vi "Dresden R2R Sputter 03.02.2018 IY24.vi"() -> ()   [LabVIEW 2009] (continued)
        n4706 = feedback #132() -> (w7120:bool)  [unwired: 1 in]
        n4707 = case shown="8" w7160 {
          tunnel: [cluster{"x":i16, "y":i16} {"x"=0, "y"=0} ("origin") cluster{"x":i16, "y":i16} {"x"=629, "y"=455} ("origin") cluster{"x":i16, "y":i16} {"x"=52, "y"=455} ("origin") cluster{"x":i16, "y":i16} {"x"=494, "y"=235} ("origin") cluster{"x":i16, "y":i16} {"x"=176, "y"=238} ("origin") cluster{"x":i16, "y":i16} {"x"=342, "y"=709} ("origin") cluster{"x":i16, "y":i16} {"x"=233, "y"=182} ("origin") cluster{"x":i16, "y":i16} {"x"=435, "y"=182} ("origin") cluster{"x":i16, "y":i16} {"x"=323, "y"=152} ("origin")] -> w7165
          tunnel: ["" ("text") "GV" ("text") "GV" ("text") "GV-BP" ("text") "GV-BP" ("text") "MG" ("text") "CST-FIX" ("text") "CST-FIX" ("text") "PET-COOL" ("text")] -> w7164
          tunnel: ["" ("DESCRIPTION") "Gate Valve" ("DESCRIPTION") "Gate Valve" ("DESCRIPTION") "Gate Valve- By Pass" ("DESCRIPTION") "Gate Valve- By Pass" ("DESCRIPTION") "MAGNETRON" ("DESCRIPTION") "Casette Fix" ("DESCRIPTION") "Casette Fix" ("DESCRIPTION") "Petfolio Cool" ("DESCRIPTION")] -> w7163
          frame #0 {
          }
          frame #1 {
          }
          frame #2 {
          }
          frame #3 {
          }
          frame #4 {
          }
          frame #5 {
          }
          frame #6 {
          }
          frame #7 {
          }
          frame #8 {
          }
        }
        n4708 = case shown="True" w7118 {
          tunnel: [TRUE FALSE] -> w7125
          tunnel: w7124 -> [_ w7209]
          frame #0 {
          }
          frame #1 {
            n4709 = call "Elapsed Time57"("Reset"=w7209) -> ("Elapsed Time (s)"=w7206:dbl)  [unwired: 11 in, 7 out]
            n4710 = Greater?(x=w7206, y=3.0) -> (0:w7207:bool)
            n4711 = In Range and Coerce(upper limit=3.0, x=w7206, lower limit=0.0) -> (In Range?=w7202:bool)  [unwired: 1 out]
            n4712 = Not(x=w7207) -> (.not. x?=w7203:bool)
            n4713 = property on="Gv_ch3_4_timer_front_gui" class="TabCtl (strict)"("Visible"=w7202) -> ()  [unwired: 2 in, 2 out]
            n4714 = local write "Gv_timer_front_ch3_4"(w7203) -> ()
          }
        }
        n4715 = case shown="True" w7093 {
          tunnel: [TRUE FALSE] -> w7122
          tunnel: w7123 -> [_ w7199]
          frame #0 {
          }
          frame #1 {
            n4716 = call "Elapsed Time58"("Reset"=w7199) -> ("Elapsed Time (s)"=w7196:dbl)  [unwired: 11 in, 7 out]
            n4717 = Greater?(x=w7196, y=3.0) -> (0:w7197:bool)
            n4718 = In Range and Coerce(upper limit=3.0, x=w7196, lower limit=0.0) -> (In Range?=w7193:bool)  [unwired: 1 out]
            n4719 = Not(x=w7197) -> (.not. x?=w7192:bool)
            n4720 = local write "Ch3_trns_gv_bp2_timer_front"(w7192) -> ()
            n4721 = property on="Ch3_trns_gv_bp2_front_gui" class="TabCtl (strict)"("Visible"=w7193) -> ()  [unwired: 2 in, 2 out]
          }
        }
        n4722 = case shown="True" w7119 {
          tunnel: [TRUE FALSE] -> w7127
          tunnel: w7126 -> [_ w7219]
          frame #0 {
          }
          frame #1 {
            n4723 = call "Elapsed Time56"("Reset"=w7219) -> ("Elapsed Time (s)"=w7216:dbl)  [unwired: 11 in, 7 out]
            n4724 = Greater?(x=w7216, y=3.0) -> (0:w7217:bool)
            n4725 = In Range and Coerce(upper limit=3.0, x=w7216, lower limit=0.0) -> (In Range?=w7212:bool)  [unwired: 1 out]
            n4726 = Not(x=w7217) -> (.not. x?=w7213:bool)
            n4727 = local write "Gv_timer_front_ch3_2"(w7213) -> ()
            n4728 = property on="Gv_ch3_2_timer_front_gui" class="TabCtl (strict)"("Visible"=w7212) -> ()  [unwired: 2 in, 2 out]
          }
        }
        n4729 = case shown="True" w7092 {
          tunnel: [TRUE FALSE] -> w7121
          tunnel: w7120 -> [_ w7189]
          frame #0 {
          }
          frame #1 {
            n4730 = call "Elapsed Time59"("Reset"=w7189) -> ("Elapsed Time (s)"=w7186:dbl)  [unwired: 11 in, 7 out]
            n4731 = Greater?(x=w7186, y=3.0) -> (0:w7187:bool)
            n4732 = In Range and Coerce(upper limit=3.0, x=w7186, lower limit=0.0) -> (In Range?=w7183:bool)  [unwired: 1 out]
            n4733 = Not(x=w7187) -> (.not. x?=w7182:bool)
            n4734 = local write "Ch3_trns_gv_bp_timer_front"(w7182) -> ()
            n4735 = property on="Ch3_trns_gv_bp_timer_front_gui" class="TabCtl (strict)"("Visible"=w7183) -> ()  [unwired: 2 in, 2 out]
          }
        }
        n4736 = local write "DESCRIPTION"(w7163) -> ()
        n4737 = call <vilib>:"Draw Text at Point.vi"("[user-specified font]"=T35 {"Font Name:"="BOLD", "Size"=18, "Strikeout?"=FALSE, "Italic?"=FALSE, "Underline?"=FALSE, "Outline?"=FALSE, "Shadow?"=FALSE, "Bold?"=TRUE} ("[user-specified font] 4"), "desired font(Application)"=T36."User-specified Font", "text"=w7164, "origin"=w7165, "picture"=w7168) -> ("new picture"=w7167:picture)  [unwired: 5 in, 1 out]
      }
    }
    "new picture 3" <- w6550
    n4738 = stacked-sequence {
      tunnel: w6559 -> [w6685 _]
      tunnel: w6560 -> [w6684 _]
      tunnel: w6561 -> [w6683 _]
      tunnel: [_ w6856] -> w6549
      tunnel: w6552 -> [w6670 _]
      tunnel: w6551 -> [w6669 _]
      tunnel: w6546 -> [w6661 _]
      tunnel: w6545 -> [w6660 _]
      tunnel: w6544 -> [w6603 _]
      tunnel: w6543 -> [w6602 _]
      tunnel: w6542 -> [w6601 _]
      tunnel: w6541 -> [w6600 _]
      tunnel: w6540 -> [w6599 _]
      tunnel: w6539 -> [w6598 _]
      tunnel: w6538 -> [w6597 _]
      tunnel: w6537 -> [w6596 _]
      tunnel: w6536 -> [w6595 _]
      tunnel: w6535 -> [w6594 _]
      tunnel: w6534 -> [w6593 _]
      tunnel: w6533 -> [w6592 _]
      tunnel: w6532 -> [w6591 _]
      tunnel: w6531 -> [w6590 _]
      tunnel: w6530 -> [w6570 _]
      tunnel: w6529 -> [w6569 _]
      frame #0 {
        n4739 = Build Array(FALSE ("element"), "chamber 3 top piston failed", "chamber 3 top piston open") -> (w6686:bool[])
        n4740 = Build Array(FALSE ("element"), "gv top open_ch3_4", "gv top failed_ch3_4") -> (w6678:bool[])
        n4741 = Build Array(FALSE ("element"), "gv top failed_ch3_2", "gv top_open_ch3_2") -> (w6662:bool[])
        n4742 = Build Array(FALSE ("element"), "ch3_atm_fail_top", "ch3_atm_on_top") -> (w6608:bool[])
        n4743 = Build Array(FALSE ("element"), "ch3_pg_fail_top", "ch3_pg_on_top") -> (w6615:bool[])
        n4744 = Build Array(FALSE ("element"), "ch3_cc_fail_top", "ch3_cc_on_top") -> (w6623:bool[])
        n4745 = Build Array(FALSE ("element"), "ch3_bg_fail_top", "ch3_bg_on_top") -> (w6630:bool[])
        n4746 = Build Array(FALSE ("element"), "ch3_bg_bv_fail_top", "ch3_bg_bv_on_top") -> (w6638:bool[])
        n4747 = Build Array(FALSE ("element"), "ch3_sov_Ar_on_top", "ch3_sov_Ar_fail_top") -> (w6654:bool[])
        n4748 = Build Array(FALSE ("element"), "ch3_trns_gv_bp_on_top", "ch3_trns_gv_bp_fail_top") -> (w6646:bool[])
        n4749 = Boolean Array To Number(Boolean array=w6686) -> (number=w6687:u32)
        n4750 = Build Array(FALSE ("element"), "ch3_trns_gv_bp2_on_top", "ch3_trns_gv_bp2_fail_top") -> (w6574:bool[])
        n4751 = Boolean Array To Number(Boolean array=w6678) -> (number=w6677:u32)
        n4752 = Boolean Array To Number(Boolean array=w6662) -> (number=w6663:u32)
        n4753 = Boolean Array To Number(Boolean array=w6608) -> (number=w6609:u32)
        n4754 = Boolean Array To Number(Boolean array=w6615) -> (number=w6614:u32)
        n4755 = Boolean Array To Number(Boolean array=w6623) -> (number=w6624:u32)
        n4756 = Boolean Array To Number(Boolean array=w6630) -> (number=w6631:u32)
        n4757 = Boolean Array To Number(Boolean array=w6638) -> (number=w6637:u32)
        n4758 = Boolean Array To Number(Boolean array=w6654) -> (number=w6653:u32)
        n4759 = Boolean Array To Number(Boolean array=w6646) -> (number=w6647:u32)
        n4760 = Boolean Array To Number(Boolean array=w6574) -> (number=w6575:u32)
        n4761 = Mantissa & Exponent(0:w6687) -> (2:w6688:dbl)  [unwired: 1 out]
        n4762 = Mantissa & Exponent(0:w6677) -> (2:w6676:dbl)  [unwired: 1 out]
        n4763 = Mantissa & Exponent(0:w6663) -> (2:w6664:dbl)  [unwired: 1 out]
        n4764 = Mantissa & Exponent(0:w6609) -> (2:w6610:dbl)  [unwired: 1 out]
        n4765 = Mantissa & Exponent(0:w6614) -> (2:w6613:dbl)  [unwired: 1 out]
        n4766 = Mantissa & Exponent(0:w6624) -> (2:w6625:dbl)  [unwired: 1 out]
        n4767 = Mantissa & Exponent(0:w6631) -> (2:w6632:dbl)  [unwired: 1 out]
        n4768 = Mantissa & Exponent(0:w6637) -> (2:w6636:dbl)  [unwired: 1 out]
        n4769 = Mantissa & Exponent(0:w6653) -> (2:w6652:dbl)  [unwired: 1 out]
        n4770 = Mantissa & Exponent(0:w6647) -> (2:w6648:dbl)  [unwired: 1 out]
        n4771 = Mantissa & Exponent(0:w6575) -> (2:w6576:dbl)  [unwired: 1 out]
        n4772 = case shown="2" w6688 {
          tunnel: [u32[][] [] ("data (RGB format)") w6723 w6725] -> w6689
          tunnel: w6684 -> [_ w6723 _]
          tunnel: w6683 -> [_ _ w6725]
          tunnel: [cluster{"x":i16, "y":i16} {"x"=0, "y"=0} ("top left point(0, 0)") cluster{"x":i16, "y":i16} {"x"=100, "y"=167} ("top left point(0, 0)") cluster{"x":i16, "y":i16} {"x"=100, "y"=168} ("top left point(0, 0)")] -> w6588
          frame #0 {
          }
          frame #1 {
          }
          frame #2 {
          }
        }
        n4773 = case shown="2" w6676 {
          tunnel: [u32[][] [] ("data (RGB format)") w6718 w6719] -> w6675
          tunnel: w6670 -> [_ w6718 _]
          tunnel: w6669 -> [_ _ w6719]
          frame #0 {
          }
          frame #1 {
          }
          frame #2 {
          }
        }
        n4774 = case shown="0, Default" w6664 {
          tunnel: [u32[][] [] ("data (RGB format)") w6715 w6716] -> w6665
          tunnel: w6661 -> [_ w6715 _]
          tunnel: w6660 -> [_ _ w6716]
          frame #0 {
          }
          frame #1 {
          }
          frame #2 {
          }
        }
        n4775 = case shown="2" w6610 {
          tunnel: w6603 -> [_ w6712 _]
          tunnel: [u32[][] [] ("data (RGB format)") w6712 w6713] -> w6611
          tunnel: w6602 -> [_ _ w6713]
          frame #0 {
          }
          frame #1 {
          }
          frame #2 {
          }
        }
        n4776 = case shown="2" w6613 {
          tunnel: w6590 -> [_ w6709 _]
          tunnel: [u32[][] [] ("data (RGB format)") w6709 w6710] -> w6612
          tunnel: w6591 -> [_ _ w6710]
          frame #0 {
          }
          frame #1 {
          }
          frame #2 {
          }
        }
        n4777 = case shown="0, Default" w6625 {
          tunnel: w6592 -> [_ w6706 _]
          tunnel: w6593 -> [_ _ w6707]
          tunnel: [u32[][] [] ("data (RGB format)") w6706 w6707] -> w6583
          frame #0 {
          }
          frame #1 {
          }
          frame #2 {
          }
        }
        n4778 = case shown="0, Default" w6632 {
          tunnel: w6601 -> [_ w6703 _]
          tunnel: [u32[][] [] ("data (RGB format)") w6703 w6704] -> w6633
          tunnel: w6600 -> [_ _ w6704]
          frame #0 {
          }
          frame #1 {
          }
          frame #2 {
          }
        }
        n4779 = case shown="2" w6636 {
          tunnel: [u32[][] [] ("data (RGB format)") w6700 w6701] -> w6635
          tunnel: w6598 -> [_ _ w6701]
          tunnel: w6599 -> [_ w6700 _]
          frame #0 {
          }
          frame #1 {
          }
          frame #2 {
          }
        }
        n4780 = case shown="0, Default" w6652 {
          tunnel: w6595 -> [_ w6694 _]
          tunnel: [u32[][] [] ("data (RGB format)") w6694 w6695] -> w6651
          tunnel: w6594 -> [_ _ w6695]
          frame #0 {
          }
          frame #1 {
          }
          frame #2 {
          }
        }
        n4781 = case shown="2" w6648 {
          tunnel: w6597 -> [_ w6697 _]
          tunnel: [u32[][] [] ("data (RGB format)") w6697 w6698] -> w6649
          tunnel: w6596 -> [_ _ w6698]
          frame #0 {
          }
          frame #1 {
          }
          frame #2 {
          }
        }
        n4782 = case shown="0, Default" w6576 {
          tunnel: w6570 -> [_ w6691 _]
          tunnel: [u32[][] [] ("data (RGB format)") w6691 w6692] -> w6577
          tunnel: w6569 -> [_ _ w6692]
          frame #0 {
          }
          frame #1 {
          }
          frame #2 {
          }
        }
        n4783 = call-poly <vilib>:"Draw Unflattened Pixmap.vi"("top left point(0, 0)"=cluster{"x":i16, "y":i16} {"x"=100, "y"=167} ("top left point(0, 0) 4"), "data (RGB format)"=w6685) -> ("new picture"=w6679:picture)  [unwired: 7 in]
        n4784 = call-poly <vilib>:"Draw Unflattened Pixmap.vi"("picture"=w6679, "top left point(0, 0)"=w6588, "data (RGB format)"=w6689) -> ("new picture"=w6674:picture)  [unwired: 6 in]
        n4785 = call-poly <vilib>:"Draw Unflattened Pixmap.vi"("picture"=w6674, "top left point(0, 0)"=cluster{"x":i16, "y":i16} {"x"=571, "y"=342} ("top left point(0, 0) 3"), "data (RGB format)"=w6675) -> ("new picture"=w6659:picture)  [unwired: 6 in]
        n4786 = call-poly <vilib>:"Draw Unflattened Pixmap.vi"("picture"=w6659, "top left point(0, 0)"=cluster{"x":i16, "y":i16} {"x"=100, "y"=342} ("top left point(0, 0) 2"), "data (RGB format)"=w6665) -> ("new picture"=w6604:picture)  [unwired: 6 in]
        n4787 = call-poly <vilib>:"Draw Unflattened Pixmap.vi"("picture"=w6604, "top left point(0, 0)"=cluster{"x":i16, "y":i16} {"x"=484, "y"=640} ("top left point(0, 0) 2"), "data (RGB format)"=w6611) -> ("new picture"=w6619:picture)  [unwired: 6 in]
        n4788 = call-poly <vilib>:"Draw Unflattened Pixmap.vi"("picture"=w6619, "top left point(0, 0)"=cluster{"x":i16, "y":i16} {"x"=204, "y"=618} ("top left point(0, 0) 2"), "data (RGB format)"=w6612) -> ("new picture"=w6626:picture)  [unwired: 6 in]
        n4789 = call-poly <vilib>:"Draw Unflattened Pixmap.vi"("picture"=w6626, "top left point(0, 0)"=cluster{"x":i16, "y":i16} {"x"=279, "y"=625} ("top left point(0, 0) 2"), "data (RGB format)"=w6583) -> ("new picture"=w6634:picture)  [unwired: 6 in]
        n4790 = call-poly <vilib>:"Draw Unflattened Pixmap.vi"("picture"=w6634, "top left point(0, 0)"=cluster{"x":i16, "y":i16} {"x"=381, "y"=673} ("top left point(0, 0) 2"), "data (RGB format)"=w6633) -> ("new picture"=w6642:picture)  [unwired: 6 in]
        n4791 = call-poly <vilib>:"Draw Unflattened Pixmap.vi"("picture"=w6642, "top left point(0, 0)"=cluster{"x":i16, "y":i16} {"x"=370, "y"=635} ("top left point(0, 0) 2"), "data (RGB format)"=w6635) -> ("new picture"=w6650:picture)  [unwired: 6 in]
        n4792 = call-poly <vilib>:"Draw Unflattened Pixmap.vi"("picture"=w6650, "top left point(0, 0)"=cluster{"x":i16, "y":i16} {"x"=494, "y"=284} ("top left point(0, 0) 2"), "data (RGB format)"=w6649) -> ("new picture"=w6658:picture)  [unwired: 6 in]
        n4793 = call-poly <vilib>:"Draw Unflattened Pixmap.vi"("picture"=w6658, "top left point(0, 0)"=cluster{"x":i16, "y":i16} {"x"=512, "y"=205} ("top left point(0, 0) 2"), "data (RGB format)"=w6651) -> ("new picture"=w6566:picture)  [unwired: 6 in]
        n4794 = call-poly <vilib>:"Draw Unflattened Pixmap.vi"("picture"=w6566, "top left point(0, 0)"=cluster{"x":i16, "y":i16} {"x"=182, "y"=282}, "data (RGB format)"=w6577) -> ("new picture"=w6567:picture)  [unwired: 6 in]
      }
      frame #1 {
        # "14"
        # "13"
        # "12"
        # "11"
        # "10"
        # "9"
        # "8"
        # "7"
        # "6"
        # "5"
        # "4"
        # "3"
        # "2"
        # "1"
        n4795 = property on="new picture 4" class="Pict"() -> ("Mouse"=w6861:T37)  [unwired: 2 in, 2 out]
        n4796 = Unbundle(w6861) -> ("Mouse Position"=w6860:cluster{"X":i32, "Y":i32}, "Mouse Modifiers"=w6868:T38)
        "Mouse Position 5" <- w6860
        n4797 = Unbundle(w6868) -> ("Button Down"=w6802:bool)  [unwired: 3 out]
        n4798 = Unbundle(w6860) -> ("X"=w6727:i32, "Y"=w6728:i32)
        n4799 = In Range and Coerce(upper limit=596, x=w6728, lower limit=359) -> (In Range?=w6850:bool)  [unwired: 1 out]
        n4800 = In Range and Coerce(upper limit=595, x=w6728, lower limit=354) -> (In Range?=w6862:bool)  [unwired: 1 out]
        n4801 = In Range and Coerce(upper limit=146, x=w6727, lower limit=106) -> (In Range?=w6849:bool)  [unwired: 1 out]
        n4802 = In Range and Coerce(upper limit=670, x=w6728, lower limit=636) -> (In Range?=w6840:bool)  [unwired: 1 out]
        n4803 = In Range and Coerce(upper limit=619, x=w6727, lower limit=579) -> (In Range?=w6863:bool)  [unwired: 1 out]
        n4804 = In Range and Coerce(upper limit=315, x=w6727, lower limit=278) -> (In Range?=w6841:bool)  [unwired: 1 out]
        n4805 = In Range and Coerce(upper limit=660, x=w6728, lower limit=636) -> (In Range?=w6839:bool)  [unwired: 1 out]
        n4806 = In Range and Coerce(upper limit=312, x=w6728, lower limit=287) -> (In Range?=w6828:bool)  [unwired: 1 out]
        n4807 = In Range and Coerce(upper limit=243, x=w6728, lower limit=198) -> (In Range?=w6733:bool)  [unwired: 1 out]
        n4808 = In Range and Coerce(upper limit=407, x=w6727, lower limit=370) -> (In Range?=w6838:bool)  [unwired: 1 out]
        n4809 = In Range and Coerce(upper limit=531, x=w6727, lower limit=493) -> (In Range?=w6829:bool)  [unwired: 1 out]
        n4810 = In Range and Coerce(upper limit=391, x=w6728, lower limit=171) -> (In Range?=w6739:bool)  [unwired: 1 out]
        n4811 = In Range and Coerce(upper limit=593, x=w6727, lower limit=564) -> (In Range?=w6732:bool)  [unwired: 1 out]
        n4812 = In Range and Coerce(upper limit=310, x=w6728, lower limit=285) -> (In Range?=w6816:bool)  [unwired: 1 out]
        n4813 = In Range and Coerce(upper limit=381, x=w6727, lower limit=339) -> (In Range?=w6740:bool)  [unwired: 1 out]
        n4814 = In Range and Coerce(upper limit=254, x=w6728, lower limit=204) -> (In Range?=w6827:bool)  [unwired: 1 out]
        n4815 = In Range and Coerce(upper limit=228, x=w6727, lower limit=191) -> (In Range?=w6817:bool)  [unwired: 1 out]
        n4816 = In Range and Coerce(upper limit=367, x=w6728, lower limit=216) -> (In Range?=w6750:bool)  [unwired: 1 out]
        n4817 = In Range and Coerce(upper limit=367, x=w6728, lower limit=216) -> (In Range?=w6749:bool)  [unwired: 1 out]
        n4818 = In Range and Coerce(upper limit=536, x=w6727, lower limit=513) -> (In Range?=w6826:bool)  [unwired: 1 out]
        n4819 = In Range and Coerce(upper limit=305, x=w6727, lower limit=255) -> (In Range?=w6751:bool)  [unwired: 1 out]
        n4820 = In Range and Coerce(upper limit=463, x=w6727, lower limit=409) -> (In Range?=w6748:bool)  [unwired: 1 out]
        n4821 = In Range and Coerce(upper limit=705, x=w6728, lower limit=682) -> (In Range?=w6789:bool)  [unwired: 1 out]
        n4822 = In Range and Coerce(upper limit=652, x=w6728, lower limit=626) -> (In Range?=w6790:bool)  [unwired: 1 out]
        n4823 = In Range and Coerce(upper limit=406, x=w6727, lower limit=381) -> (In Range?=w6788:bool)  [unwired: 1 out]
        n4824 = In Range and Coerce(upper limit=229, x=w6727, lower limit=204) -> (In Range?=w6791:bool)  [unwired: 1 out]
        n4825 = In Range and Coerce(upper limit=674, x=w6728, lower limit=648) -> (In Range?=w6756:bool)  [unwired: 1 out]
        n4826 = In Range and Coerce(upper limit=530, x=w6727, lower limit=484) -> (In Range?=w6800:bool)  [unwired: 1 out]
        n4827 = And(x=w6849, y=w6850) -> (x .and. y?=w6812:bool)
        n4828 = And(x=w6863, y=w6862) -> (x .and. y?=w6813:bool)
        n4829 = And(x=w6841, y=w6840) -> (x .and. y?=w6811:bool)
        n4830 = And(x=w6838, y=w6839) -> (x .and. y?=w6810:bool)
        n4831 = And(x=w6829, y=w6828) -> (x .and. y?=w6808:bool)
        n4832 = And(x=w6732, y=w6733) -> (x .and. y?=w6726:bool)
        n4833 = And(x=w6740, y=w6739) -> (x .and. y?=w6736:bool)
        n4834 = And(x=w6817, y=w6816) -> (x .and. y?=w6779:bool)
        n4835 = And(x=w6826, y=w6827) -> (x .and. y?=w6809:bool)
        n4836 = And(x=w6751, y=w6750) -> (x .and. y?=w6738:bool)
        n4837 = And(x=w6748, y=w6749) -> (x .and. y?=w6737:bool)
        n4838 = And(x=w6788, y=w6789) -> (x .and. y?=w6781:bool)
        n4839 = And(x=w6791, y=w6790) -> (x .and. y?=w6782:bool)
        n4840 = And(x=w6800, y=w6756) -> (x .and. y?=w6783:bool)
        n4841 = And(x=w6802, y=w6812) -> (x .and. y?=w6807:bool)
        n4842 = And(x=w6802, y=w6813) -> (x .and. y?=w6815:bool)
        n4843 = And(x=w6802, y=w6811) -> (x .and. y?=w6806:bool)
        n4844 = And(x=w6802, y=w6810) -> (x .and. y?=w6805:bool)
        n4845 = And(x=w6802, y=w6808) -> (x .and. y?=w6804:bool)
        n4846 = And(x=w6802, y=w6779) -> (x .and. y?=w6778:bool)
        n4847 = And(x=w6802, y=w6809) -> (x .and. y?=w6803:bool)
        n4848 = case shown="True" w6807 {
          frame #0 {
          }
          frame #1 {
            "gv_top_timer_ch3_4" <- TRUE ("gv_top_timer_ch2_12")
          }
        }
        n4849 = case shown="True" w6815 {
          frame #0 {
          }
          frame #1 {
            "gv_top_timer_ch3_2" <- TRUE ("gv_top_timer_ch2_3")
          }
        }
        n4850 = case shown="True" w6806 {
          frame #0 {
          }
          frame #1 {
            "ch3_cc_timer_top" <- TRUE ("ch2_cc_timer_top")
          }
        }
        n4851 = case shown="True" w6805 {
          frame #0 {
          }
          frame #1 {
            "ch3_bg_bv_timer_top" <- TRUE ("ch2_cc_timer_top")
          }
        }
        n4852 = case shown="True" w6804 {
          frame #0 {
          }
          frame #1 {
            "ch3_trns_gv_bp_timer_top" <- TRUE ("ch2_cc_timer_top")
          }
        }
        n4853 = case shown="True" w6778 {
          frame #0 {
          }
          frame #1 {
            "ch3_trns_gv_bp2_timer_top" <- TRUE ("ch2_cc_timer_top")
          }
        }
        n4854 = case shown="True" w6803 {
          frame #0 {
          }
          frame #1 {
            "ch3_sov_Ar_timer_top" <- TRUE ("ch2_cc_timer_top")
          }
        }
        n4855 = Build Array(TRUE, w6813, w6812, w6811, w6810, w6808, w6809, w6779, w6783, w6782, w6781, w6738, w6737, w6736, w6726) -> (w6780:bool[])
        n4856 = local read "ch3_trns_gv_bp_timer_top"() -> (w6759:bool)
        n4857 = local read "ch3_trns_gv_bp2_timer_top"() -> (w6758:bool)
        n4858 = local read "gv_top_timer_ch3_4"() -> (w6762:bool)
        n4859 = local read "ch3_bg_bv_timer_top"() -> (w6760:bool)
        n4860 = local read "ch3_sov_Ar_timer_top"() -> (w6757:bool)
        n4861 = local read "gv_top_timer_ch3_2"() -> (w6763:bool)
        n4862 = local read "ch3_cc_timer_top"() -> (w6761:bool)
        n4863 = Boolean Array To Number(Boolean array=w6780) -> (number=w6859:u32)
        n4864 = Mantissa & Exponent(0:w6859) -> (2:w6858:dbl)  [unwired: 1 out]
        n4865 = feedback #133() -> (w6776:bool)  [unwired: 1 in]
        n4866 = feedback #134() -> (w6774:bool)  [unwired: 1 in]
        n4867 = feedback #135() -> (w6773:bool)  [unwired: 1 in]
        n4868 = feedback #136() -> (w6770:bool)  [unwired: 1 in]
        n4869 = feedback #137() -> (w6769:bool)  [unwired: 1 in]
        n4870 = feedback #138() -> (w6766:bool)  [unwired: 1 in]
        n4871 = feedback #139() -> (w6765:bool)  [unwired: 1 in]
        n4872 = case shown="12" w6858 {
          tunnel: [cluster{"x":i16, "y":i16} {"x"=0, "y"=0} ("origin") cluster{"x":i16, "y":i16} {"x"=633, "y"=472} ("origin") cluster{"x":i16, "y":i16} {"x"=73, "y"=465} ("origin") cluster{"x":i16, "y":i16} {"x"=281, "y"=678} ("origin") cluster{"x":i16, "y":i16} {"x"=413, "y"=647} ("origin") cluster{"x":i16, "y":i16} {"x"=511, "y"=270} ("origin") cluster{"x":i16, "y":i16} {"x"=507, "y"=187} ("origin") cluster{"x":i16, "y":i16} {"x"=186, "y"=268} ("origin") cluster{"x":i16, "y":i16} {"x"=490, "y"=686} ("origin") cluster{"x":i16, "y":i16} {"x"=209, "y"=659} ("origin") cluster{"x":i16, "y":i16} {"x"=380, "y"=716} ("origin") cluster{"x":i16, "y":i16} {"x"=257, "y"=167} ("origin") cluster{"x":i16, "y":i16} {"x"=411, "y"=167} ("origin") cluster{"x":i16, "y":i16} {"x"=329, "y"=149} ("origin") cluster{"x":i16, "y":i16} {"x"=560, "y"=180} ("origin")] -> w6853
          tunnel: ["" ("text") "GV" ("text") "GV" ("text") "CH-CC" ("text") "BG-BV" ("text") "GV-BP" ("text") "SOV-Ar" ("text") "GV-BP" ("text") "CH-ATM" ("text") "CH-PG" ("text") "CH-BG" ("text") "CST-FIX" ("text") "CST-FIX" ("text") "PET-COOL" ("text") "MFC" ("text")] -> w6852
          tunnel: ["" ("DESCRIPTION") "Gate Valve" ("DESCRIPTION") "Gate Valve" ("DESCRIPTION") "Chamber-Cold Cathode" ("DESCRIPTION") "Baratron Gauge-Block Valve" ("DESCRIPTION") "Gate Valve- By Pass" ("DESCRIPTION") "Shut Off Valve-Ar Gas" ("DESCRIPTION") "Gate Valve- By Pass" ("DESCRIPTION") "Chamber-Atmospheric Switch" ("DESCRIPTION") "Chamber-Pirani Gauge" ("DESCRIPTION") "Chamber-Baratron Gauge" ("DESCRIPTION") "Casette Fix" ("DESCRIPTION") "Casette Fix" ("DESCRIPTION") "Petfolio Cool " ("DESCRIPTION") "Mass Flow Control" ("DESCRIPTION")] -> w6851
          frame #0 {
          }
          frame #1 {
          }
          frame #2 {
          }
          frame #3 {
          }
          frame #4 {
          }
          frame #5 {
          }
          frame #6 {
          }
          frame #7 {
          }
          frame #8 {
          }
          frame #9 {
          }
          frame #10 {
          }
          frame #11 {
          }
          frame #12 {
          }
          frame #13 {
          }
          frame #14 {
          }
        }
        n4873 = case shown="True" w6763 {
          tunnel: [TRUE FALSE] -> w6777
          tunnel: w6776 -> [_ w6937]
          frame #0 {
          }
          frame #1 {
            n4874 = call "Elapsed Time60"("Reset"=w6937) -> ("Elapsed Time (s)"=w6934:dbl)  [unwired: 11 in, 7 out]
            n4875 = Greater?(x=w6934, y=3.0) -> (0:w6935:bool)
            n4876 = In Range and Coerce(upper limit=3.0, x=w6934, lower limit=0.0) -> (In Range?=w6930:bool)  [unwired: 1 out]
            n4877 = Not(x=w6935) -> (.not. x?=w6931:bool)
            n4878 = local write "gv_top_timer_ch3_2"(w6931) -> ()
            n4879 = property on="Gv_timer_top_ch3_2_gui" class="TabCtl (strict)"("Visible"=w6930) -> ()  [unwired: 2 in, 2 out]
          }
        }
        n4880 = case shown="True" w6762 {
          tunnel: [TRUE FALSE] -> w6775
          tunnel: w6774 -> [_ w6927]
          frame #0 {
          }
          frame #1 {
            n4881 = call "Elapsed Time61"("Reset"=w6927) -> ("Elapsed Time (s)"=w6924:dbl)  [unwired: 11 in, 7 out]
            n4882 = Greater?(x=w6924, y=3.0) -> (0:w6925:bool)
            n4883 = In Range and Coerce(upper limit=3.0, x=w6924, lower limit=0.0) -> (In Range?=w6920:bool)  [unwired: 1 out]
            n4884 = Not(x=w6925) -> (.not. x?=w6921:bool)
            n4885 = local write "gv_top_timer_ch3_4"(w6921) -> ()
            n4886 = property on="Gv_timer_top_ch3_4_gui" class="TabCtl (strict)"("Visible"=w6920) -> ()  [unwired: 2 in, 2 out]
          }
        }
        n4887 = case shown="True" w6761 {
          tunnel: [TRUE FALSE] -> w6772
          tunnel: w6773 -> [_ w6917]
          frame #0 {
          }
          frame #1 {
            n4888 = call "Elapsed Time62"("Reset"=w6917) -> ("Elapsed Time (s)"=w6914:dbl)  [unwired: 11 in, 7 out]
            n4889 = Greater?(x=w6914, y=3.0) -> (0:w6915:bool)
            n4890 = In Range and Coerce(upper limit=3.0, x=w6914, lower limit=0.0) -> (In Range?=w6910:bool)  [unwired: 1 out]
            n4891 = Not(x=w6915) -> (.not. x?=w6911:bool)
            n4892 = local write "ch3_cc_timer_top"(w6911) -> ()
            n4893 = property on="Ch3_cc_timer_top_gui" class="TabCtl (strict)"("Visible"=w6910) -> ()  [unwired: 2 in, 2 out]
          }
        }
        n4894 = case shown="True" w6760 {
          tunnel: [TRUE FALSE] -> w6771
          tunnel: w6770 -> [_ w6907]
          frame #0 {
          }
          frame #1 {
            n4895 = call "Elapsed Time63"("Reset"=w6907) -> ("Elapsed Time (s)"=w6904:dbl)  [unwired: 11 in, 7 out]
            n4896 = Greater?(x=w6904, y=3.0) -> (0:w6905:bool)
            n4897 = In Range and Coerce(upper limit=3.0, x=w6904, lower limit=0.0) -> (In Range?=w6900:bool)  [unwired: 1 out]
            n4898 = Not(x=w6905) -> (.not. x?=w6901:bool)
            n4899 = local write "ch3_bg_bv_timer_top"(w6901) -> ()
            n4900 = property on="Ch3_bg_bv_timer_top_gui" class="TabCtl (strict)"("Visible"=w6900) -> ()  [unwired: 2 in, 2 out]
          }
        }
        n4901 = case shown="True" w6759 {
          tunnel: [TRUE FALSE] -> w6768
          tunnel: w6769 -> [_ w6897]
          frame #0 {
          }
          frame #1 {
            n4902 = call "Elapsed Time64"("Reset"=w6897) -> ("Elapsed Time (s)"=w6894:dbl)  [unwired: 11 in, 7 out]
            n4903 = Greater?(x=w6894, y=3.0) -> (0:w6895:bool)
            n4904 = In Range and Coerce(upper limit=3.0, x=w6894, lower limit=0.0) -> (In Range?=w6890:bool)  [unwired: 1 out]
            n4905 = Not(x=w6895) -> (.not. x?=w6891:bool)
            n4906 = local write "ch3_trns_gv_bp_timer_top"(w6891) -> ()
            n4907 = property on="Ch3_trns_gv_bp_timer_top_gui" class="TabCtl (strict)"("Visible"=w6890) -> ()  [unwired: 2 in, 2 out]
          }
        }
        n4908 = case shown="True" w6758 {
          tunnel: [TRUE FALSE] -> w6767
          tunnel: w6766 -> [_ w6887]
          frame #0 {
          }
          frame #1 {
            n4909 = call "Elapsed Time65"("Reset"=w6887) -> ("Elapsed Time (s)"=w6884:dbl)  [unwired: 11 in, 7 out]
            n4910 = Greater?(x=w6884, y=3.0) -> (0:w6885:bool)
            n4911 = In Range and Coerce(upper limit=3.0, x=w6884, lower limit=0.0) -> (In Range?=w6880:bool)  [unwired: 1 out]
            n4912 = Not(x=w6885) -> (.not. x?=w6881:bool)
            n4913 = local write "ch3_trns_gv_bp2_timer_top"(w6881) -> ()
            n4914 = property on="Ch3_trns_gv_bp2_timer_top_gui" class="TabCtl (strict)"("Visible"=w6880) -> ()  [unwired: 2 in, 2 out]
          }
        }
        n4915 = case shown="True" w6757 {
          tunnel: [TRUE FALSE] -> w6764
          tunnel: w6765 -> [_ w6877]
          frame #0 {
          }
          frame #1 {
            n4916 = call "Elapsed Time66"("Reset"=w6877) -> ("Elapsed Time (s)"=w6874:dbl)  [unwired: 11 in, 7 out]
            n4917 = Greater?(x=w6874, y=3.0) -> (0:w6875:bool)
            n4918 = In Range and Coerce(upper limit=3.0, x=w6874, lower limit=0.0) -> (In Range?=w6870:bool)  [unwired: 1 out]
            n4919 = Not(x=w6875) -> (.not. x?=w6871:bool)
            n4920 = property on="Ch3_sov_Ar_timer_top_gui" class="TabCtl (strict)"("Visible"=w6870) -> ()  [unwired: 2 in, 2 out]
            n4921 = local write "ch3_sov_Ar_timer_top"(w6871) -> ()
          }
        }
        n4922 = local write "DESCRIPTION"(w6851) -> ()
        n4923 = call <vilib>:"Draw Text at Point.vi"("[user-specified font]"=T35 {"Font Name:"="BOLD", "Size"=18, "Strikeout?"=FALSE, "Italic?"=FALSE, "Underline?"=FALSE, "Outline?"=FALSE, "Shadow?"=FALSE, "Bold?"=TRUE} ("[user-specified font] 5"), "desired font(Application)"=T36."User-specified Font", "text"=w6852, "origin"=w6853, "picture"=w6857) -> ("new picture"=w6856:picture)  [unwired: 5 in, 1 out]
      }
    }
    "new picture 4" <- w6549
    n4924 = Wait Until Next ms Multiple(millisecond multiple=u32 100) -> ()  [unwired: 1 out]
  }
  n4925 = while {
    tunnel: w370 -> [w7282]
    tunnel: w371 -> [w7283]
    tunnel: w372 -> [w7281]
    tunnel: w373 -> [w7280]
    tunnel: w374 -> [w7279]
    tunnel: w375 -> [w7278]
    tunnel: w376 -> [w7277]
    tunnel: w377 -> [w7276]
    tunnel: w378 -> [w7275]
    tunnel: w379 -> [w7274]
    tunnel: w380 -> [w7273]
    tunnel: w381 -> [w7272]
    tunnel: w382 -> [w7271]
    tunnel: w383 -> [w7270]
    tunnel: w101 -> [w7268]
    tunnel: w100 -> [w7267]
    tunnel: w92 -> [w7266]
    tunnel: w91 -> [w7265]
    tunnel: w60 -> [w7264]
    tunnel: w59 -> [w7263]
    tunnel: w58 -> [w7262]
    tunnel: w57 -> [w7261]
    tunnel: w56 -> [w7260]
    tunnel: w55 -> [w7259]
    tunnel: w54 -> [w7258]
    tunnel: w53 -> [w7257]
    tunnel: w52 -> [w7256]
    tunnel: w51 -> [w7255]
    tunnel: w34 -> [w7253]
    tunnel: w33 -> [w7252]
    stop <- FALSE stop-if-true
    n4926 = Wait Until Next ms Multiple(millisecond multiple=u32 100) -> ()  [unwired: 1 out]
    n4927 = stacked-sequence {
      tunnel: w7283 -> [w7387 _]
      tunnel: w7273 -> [w7382 _]
      tunnel: w7272 -> [w7381 _]
      tunnel: w7271 -> [w7369 _]
      tunnel: w7270 -> [w7368 _]
      tunnel: w7266 -> [w7355 _]
      tunnel: w7265 -> [w7354 _]
      tunnel: w7264 -> [w7329 _]
      tunnel: w7263 -> [w7328 _]
      tunnel: w7262 -> [w7327 _]
      tunnel: w7261 -> [w7326 _]
      tunnel: w7260 -> [w7325 _]
      tunnel: w7259 -> [w7324 _]
      tunnel: w7258 -> [w7323 _]
      tunnel: w7257 -> [w7298 _]
      tunnel: w7256 -> [w7322 _]
      tunnel: w7255 -> [w7321 _]
      tunnel: [_ w7522] -> w7254
      tunnel: w7253 -> [w7291 _]
      tunnel: w7252 -> [w7290 _]
      frame #0 {
        n4928 = Build Array(FALSE ("element"), "ch1_pg_fail_top", "ch1_pg_on_top") -> (w7307:bool[])
        n4929 = Build Array(FALSE ("element"), "ch1_cc_fail_top", "ch1_cc_on_top") -> (w7314:bool[])
        n4930 = Build Array(FALSE ("element"), "ch1_bg_fail_top", "ch1_bg_on_top") -> (w7300:bool[])
        n4931 = Build Array(FALSE ("element"), "gv top open ch1", "gv top failed ch1") -> (w7374:bool[])
        n4932 = Build Array(FALSE ("element"), "ch1_bg_bv_fail_top", "ch1_bg_bv_on_top") -> (w7299:bool[])
        n4933 = Build Array(FALSE ("element"), "ch1_sov_Ar_on_top", "ch1_sov_Ar_fail_top") -> (w7297:bool[])
        n4934 = Build Array(FALSE ("element"), "chamber 1 top piston open ch1", "chamber 1 top piston failed ch1") -> (w7386:bool[])
        n4935 = Build Array(FALSE ("element"), "Trns_gv_bp2_ch1_fail_top", "Trns_gv_bp2_ch1_on_top") -> (w7357:bool[])
        n4936 = Build Array(FALSE ("element"), "ch1_atm_fail_top", "ch1_atm_on_top") -> (w7302:bool[])
        n4937 = Boolean Array To Number(Boolean array=w7307) -> (number=w7306:u32)
        n4938 = Boolean Array To Number(Boolean array=w7314) -> (number=w7301:u32)
        n4939 = Boolean Array To Number(Boolean array=w7374) -> (number=w7375:u32)
        n4940 = Boolean Array To Number(Boolean array=w7386) -> (number=w7385:u32)
        n4941 = Boolean Array To Number(Boolean array=w7357) -> (number=w7358:u32)
        n4942 = Boolean Array To Number(Boolean array=w7302) -> (number=w7353:u32)
        n4943 = Boolean Array To Number(Boolean array=w7300) -> (number=w7340:u32)
        n4944 = Boolean Array To Number(Boolean array=w7299) -> (number=w7339:u32)
        n4945 = Boolean Array To Number(Boolean array=w7297) -> (number=w7296:u32)
        n4946 = Mantissa & Exponent(0:w7375) -> (2:w7376:dbl)  [unwired: 1 out]
        n4947 = Mantissa & Exponent(0:w7385) -> (2:w7384:dbl)  [unwired: 1 out]
        n4948 = Mantissa & Exponent(0:w7358) -> (2:w7361:dbl)  [unwired: 1 out]
        n4949 = Mantissa & Exponent(0:w7353) -> (2:w7352:dbl)  [unwired: 1 out]
        n4950 = Mantissa & Exponent(0:w7301) -> (2:w7346:dbl)  [unwired: 1 out]
        n4951 = Mantissa & Exponent(0:w7306) -> (2:w7347:dbl)  [unwired: 1 out]
        n4952 = Mantissa & Exponent(0:w7340) -> (2:w7341:dbl)  [unwired: 1 out]
        n4953 = Mantissa & Exponent(0:w7339) -> (2:w7338:dbl)  [unwired: 1 out]
        n4954 = Mantissa & Exponent(0:w7296) -> (2:w7292:dbl)  [unwired: 1 out]
        n4955 = case shown="2" w7376 {
          tunnel: w7368 -> [_ w7410 _]
          tunnel: [u32[][] [] ("data (RGB format)") w7410 w7411] -> w7377
          tunnel: w7369 -> [_ _ w7411]
          frame #0 {
          }
          frame #1 {
          }
          frame #2 {
          }
        }
        n4956 = case shown="2" w7384 {
          tunnel: w7381 -> [_ w7413 _]
          tunnel: [u32[][] [] ("data (RGB format)") w7413 w7414] -> w7383
          tunnel: w7382 -> [_ _ w7414]
          frame #0 {
          }
          frame #1 {
          }
          frame #2 {
          }
        }
        n4957 = case shown="0, Default" w7361 {
          tunnel: w7355 -> [_ w7407 _]
          tunnel: [u32[][] [] ("data (RGB format)") w7407 w7408] -> w7362
          tunnel: w7354 -> [_ _ w7408]
          frame #0 {
          }
          frame #1 {
          }
          frame #2 {
          }
        }
        n4958 = case shown="0, Default" w7352 {
          tunnel: w7329 -> [_ w7404 _]
          tunnel: [u32[][] [] ("data (RGB format)") w7404 w7405] -> w7351
          tunnel: w7328 -> [_ _ w7405]
          frame #0 {
          }
          frame #1 {
          }
          frame #2 {
          }
        }
        n4959 = case shown="0, Default" w7346 {
          tunnel: w7325 -> [_ w7398 _]
          tunnel: [u32[][] [] ("data (RGB format)") w7398 w7399] -> w7345
          tunnel: w7324 -> [_ _ w7399]
          frame #0 {
          }
          frame #1 {
          }
          frame #2 {
          }
        }
        n4960 = case shown="0, Default" w7347 {
          tunnel: w7327 -> [_ w7401 _]
          tunnel: [u32[][] [] ("data (RGB format)") w7401 w7402] -> w7348
          tunnel: w7326 -> [_ _ w7402]
          frame #0 {
          }
          frame #1 {
          }
          frame #2 {
          }
        }
        n4961 = case shown="2" w7341 {
          tunnel: w7323 -> [_ w7395 _]
          tunnel: [u32[][] [] ("data (RGB format)") w7395 w7396] -> w7342
          tunnel: w7298 -> [_ _ w7396]
          frame #0 {
          }
          frame #1 {
          }
          frame #2 {
          }
        }
        n4962 = case shown="1" w7292 {
          tunnel: w7291 -> [_ w7389 _]
          tunnel: [u32[][] [] ("data (RGB format)") w7389 w7390] -> w7288
          tunnel: w7290 -> [_ _ w7390]
          frame #0 {
          }
          frame #1 {
          }
          frame #2 {
          }
        }
        n4963 = case shown="2" w7338 {
          tunnel: w7322 -> [_ w7392 _]
          tunnel: [u32[][] [] ("data (RGB format)") w7392 w7393] -> w7337
          tunnel: w7321 -> [_ _ w7393]
          frame #0 {
          }
          frame #1 {
          }
          frame #2 {
          }
        }
        n4964 = call-poly <vilib>:"Draw Unflattened Pixmap.vi"("top left point(0, 0)"=cluster{"x":i16, "y":i16} {"x"=100, "y"=167} ("top left point(0, 0) 4"), "data (RGB format)"=w7387) -> ("new picture"=w7367:picture)  [unwired: 7 in]
        n4965 = call-poly <vilib>:"Draw Unflattened Pixmap.vi"("picture"=w7367, "top left point(0, 0)"=cluster{"x":i16, "y":i16} {"x"=148, "y"=167}, "data (RGB format)"=w7383) -> ("new picture"=w7373:picture)  [unwired: 6 in]
        n4966 = call-poly <vilib>:"Draw Unflattened Pixmap.vi"("picture"=w7373, "top left point(0, 0)"=cluster{"x":i16, "y":i16} {"x"=100, "y"=343}, "data (RGB format)"=w7377) -> ("new picture"=w7335:picture)  [unwired: 6 in]
        n4967 = call-poly <vilib>:"Draw Unflattened Pixmap.vi"("picture"=w7335, "top left point(0, 0)"=cluster{"x":i16, "y":i16} {"x"=181, "y"=284}, "data (RGB format)"=w7362) -> ("new picture"=w7334:picture)  [unwired: 6 in]
        n4968 = call-poly <vilib>:"Draw Unflattened Pixmap.vi"("picture"=w7334, "top left point(0, 0)"=cluster{"x":i16, "y":i16} {"x"=484, "y"=640}, "data (RGB format)"=w7351) -> ("new picture"=w7333:picture)  [unwired: 6 in]
        n4969 = call-poly <vilib>:"Draw Unflattened Pixmap.vi"("picture"=w7333, "top left point(0, 0)"=cluster{"x":i16, "y":i16} {"x"=204, "y"=618}, "data (RGB format)"=w7348) -> ("new picture"=w7332:picture)  [unwired: 6 in]
        n4970 = call-poly <vilib>:"Draw Unflattened Pixmap.vi"("picture"=w7332, "top left point(0, 0)"=cluster{"x":i16, "y":i16} {"x"=279, "y"=623}, "data (RGB format)"=w7345) -> ("new picture"=w7331:picture)  [unwired: 6 in]
        n4971 = call-poly <vilib>:"Draw Unflattened Pixmap.vi"("picture"=w7331, "top left point(0, 0)"=cluster{"x":i16, "y":i16} {"x"=381, "y"=672}, "data (RGB format)"=w7342) -> ("new picture"=w7330:picture)  [unwired: 6 in]
        n4972 = call-poly <vilib>:"Draw Unflattened Pixmap.vi"("picture"=w7330, "top left point(0, 0)"=cluster{"x":i16, "y":i16} {"x"=370, "y"=635}, "data (RGB format)"=w7337) -> ("new picture"=w7286:picture)  [unwired: 6 in]
        n4973 = call-poly <vilib>:"Draw Unflattened Pixmap.vi"("picture"=w7286, "top left point(0, 0)"=cluster{"x":i16, "y":i16} {"x"=511, "y"=203}, "data (RGB format)"=w7288) -> ("new picture"=w7287:picture)  [unwired: 6 in]
      }
      frame #1 {
        # "9 mfc"
        # "8 sov-ar"
        # "5"
        # "6"
        # "7"
        n4974 = property on="new picture 7" class="Pict"() -> ("Mouse"=w7534:T37)  [unwired: 2 in, 2 out]
        n4975 = Unbundle(w7534) -> ("Mouse Position"=w7533:cluster{"X":i32, "Y":i32}, "Mouse Modifiers"=w7535:T38)
        "Mouse Position 9" <- w7533
        n4976 = Unbundle(w7533) -> ("X"=w7418:i32, "Y"=w7419:i32)
        n4977 = Unbundle(w7535) -> ("Button Down"=w7444:bool)  [unwired: 3 out]
        n4978 = In Range and Coerce(upper limit=662, x=w7419, lower limit=629) -> (In Range?=w7504:bool)  [unwired: 1 out]
        n4979 = In Range and Coerce(upper limit=407, x=w7418, lower limit=371) -> (In Range?=w7505:bool)  [unwired: 1 out]
        n4980 = In Range and Coerce(upper limit=243, x=w7419, lower limit=198) -> (In Range?=w7450:bool)  [unwired: 1 out]
        n4981 = In Range and Coerce(upper limit=368, x=w7419, lower limit=213) -> (In Range?=w7431:bool)  [unwired: 1 out]
        n4982 = In Range and Coerce(upper limit=670, x=w7419, lower limit=636) -> (In Range?=w7515:bool)  [unwired: 1 out]
        n4983 = In Range and Coerce(upper limit=703, x=w7419, lower limit=682) -> (In Range?=w7491:bool)  [unwired: 1 out]
        n4984 = In Range and Coerce(upper limit=255, x=w7419, lower limit=202) -> (In Range?=w7452:bool)  [unwired: 1 out]
        n4985 = In Range and Coerce(upper limit=592, x=w7418, lower limit=564) -> (In Range?=w7449:bool)  [unwired: 1 out]
        n4986 = In Range and Coerce(upper limit=461, x=w7418, lower limit=410) -> (In Range?=w7430:bool)  [unwired: 1 out]
        n4987 = In Range and Coerce(upper limit=315, x=w7418, lower limit=279) -> (In Range?=w7514:bool)  [unwired: 1 out]
        n4988 = In Range and Coerce(upper limit=409, x=w7418, lower limit=381) -> (In Range?=w7490:bool)  [unwired: 1 out]
        n4989 = In Range and Coerce(upper limit=535, x=w7418, lower limit=512) -> (In Range?=w7453:bool)  [unwired: 1 out]
        n4990 = In Range and Coerce(upper limit=313, x=w7419, lower limit=287) -> (In Range?=w7480:bool)  [unwired: 1 out]
        n4991 = In Range and Coerce(upper limit=651, x=w7419, lower limit=627) -> (In Range?=w7492:bool)  [unwired: 1 out]
        n4992 = In Range and Coerce(upper limit=361, x=w7419, lower limit=170) -> (In Range?=w7420:bool)  [unwired: 1 out]
        n4993 = In Range and Coerce(upper limit=227, x=w7418, lower limit=191) -> (In Range?=w7479:bool)  [unwired: 1 out]
        n4994 = In Range and Coerce(upper limit=233, x=w7418, lower limit=206) -> (In Range?=w7493:bool)  [unwired: 1 out]
        n4995 = In Range and Coerce(upper limit=368, x=w7419, lower limit=213) -> (In Range?=w7432:bool)  [unwired: 1 out]
        n4996 = In Range and Coerce(upper limit=381, x=w7418, lower limit=338) -> (In Range?=w7421:bool)  [unwired: 1 out]
        n4997 = In Range and Coerce(upper limit=676, x=w7419, lower limit=646) -> (In Range?=w7503:bool)  [unwired: 1 out]
        n4998 = In Range and Coerce(upper limit=306, x=w7418, lower limit=258) -> (In Range?=w7433:bool)  [unwired: 1 out]
        n4999 = In Range and Coerce(upper limit=530, x=w7418, lower limit=486) -> (In Range?=w7502:bool)  [unwired: 1 out]
        n5000 = In Range and Coerce(upper limit=595, x=w7419, lower limit=355) -> (In Range?=w7516:bool)  [unwired: 1 out]
        n5001 = In Range and Coerce(upper limit=144, x=w7418, lower limit=106) -> (In Range?=w7517:bool)  [unwired: 1 out]
        n5002 = And(x=w7505, y=w7504) -> (x .and. y?=w7472:bool)
        n5003 = And(x=w7449, y=w7450) -> (x .and. y?=w7443:bool)
        n5004 = And(x=w7430, y=w7431) -> (x .and. y?=w7416:bool)
        n5005 = And(x=w7514, y=w7515) -> (x .and. y?=w7473:bool)
        n5006 = And(x=w7490, y=w7491) -> (x .and. y?=w7451:bool)
        n5007 = And(x=w7453, y=w7452) -> (x .and. y?=w7439:bool)
        n5008 = And(x=w7479, y=w7480) -> (x .and. y?=w7474:bool)
        n5009 = And(x=w7493, y=w7492) -> (x .and. y?=w7470:bool)
        n5010 = And(x=w7421, y=w7420) -> (x .and. y?=w7415:bool)
        n5011 = And(x=w7433, y=w7432) -> (x .and. y?=w7417:bool)
        n5012 = And(x=w7502, y=w7503) -> (x .and. y?=w7471:bool)
        n5013 = And(x=w7517, y=w7516) -> (x .and. y?=w7484:bool)
        n5014 = And(x=w7444, y=w7474) -> (x .and. y?=w7481:bool)
        n5015 = And(x=w7444, y=w7472) -> (x .and. y?=w7482:bool)
        n5016 = And(x=w7444, y=w7473) -> (x .and. y?=w7483:bool)
        n5017 = And(x=w7444, y=w7484) -> (x .and. y?=w7485:bool)
        n5018 = And(x=w7444, y=w7439) -> (x .and. y?=w7438:bool)